vi "CalibrateCameraHeight (Standalone).vi"(0 "Inputs: Collect Images":T4={"Image feed"=refnum, "Axes Speeds [mm/s]"={"X Speed"=10.0, "Y Speed"=10.0, "Z Speed"=10.0}, "XYZ .NET Refnum in"=refnum}, 2 "Autofocus Coordinates":T3, 3 "Focusing test range [mm]":dbl, 4 "Stepsize [mm]":dbl, 5 "error in (no error)":errorcluster, 8 "Path to save collected images":path=path "E:/XYZstage+Camera_CollectedImages/12-17-2016/images") -> (14 "Optimized working distance [mm]":dbl, 15 "Uncertainty on optimized Z [mm]":dbl, 19 "error out":errorcluster)   [LabVIEW 2016]
uses:
  C:/Users/Aerotech/Documents/BNLStaveAssembly-blueprint/Bin/Aerotech.A3200.dll
  BNLStaveAssembly-blueprint/Bin/Aerotech.A3200.dll
  <vilib>/userdefined/High Color/IMAQdx.ctl
  <vilib>/vision/Image Controls.llb/IMAQ Image.ctl
  AerotechLibraries/Motion/EnableMultiple.vi
  <vilib>/vision/driver/NI_Vision_Acquisition_Software.lvlib
panel:
  in  "Wait time before \nimage capture [s]":dbl=3.5
  out "Wait to capture [ms]":u32=3500
  out "VISA error out":errorcluster
  out "double( Time, Temp )":dbl[](array[numeric])
  in  "stop":bool
  out "Camera error out":errorcluster
  in  "Camera gain":dbl=16.0
  out "Current field of view":T1(plugin-control)
  in  "Camera Name":T2="cam1" caption="IMAQdx Session"
  in  "Tab Control":enum32{"Inputs", "Results", "Error handling"}(tab)
  in  "Si Gain":dbl=9.5 format="%#_13g"
  in  "Spotlight":bool
  in  "Stave Gain":dbl=16.0 format="%#_13g"
  # "CALIBRATE CAMERA HEIGHT Brandeis University - Brookhaven National Laboratory * ATLAS Phase II Inner Tracker Upgrade"
types:
  T1 = typedef "IMAQ Image.ctl" = refnum<image>
  T2 = typedef "IMAQdx.ctl" = refnum<k21>
  T3 = cluster{"Go to X":dbl, "Go to Y":dbl, "Go to Z":dbl}
  T4 = cluster{"Image feed":T1, "Axes Speeds [mm/s]":cluster{"X Speed":dbl, "Y Speed":dbl, "Z Speed":dbl}, "XYZ .NET Refnum in":refnum<k24>}
  T5 = typedef "Image Type" = u32
  T6 = cluster{"Captured positions":dbl[][], "XYZ .NET Refnum out":refnum<k24>}
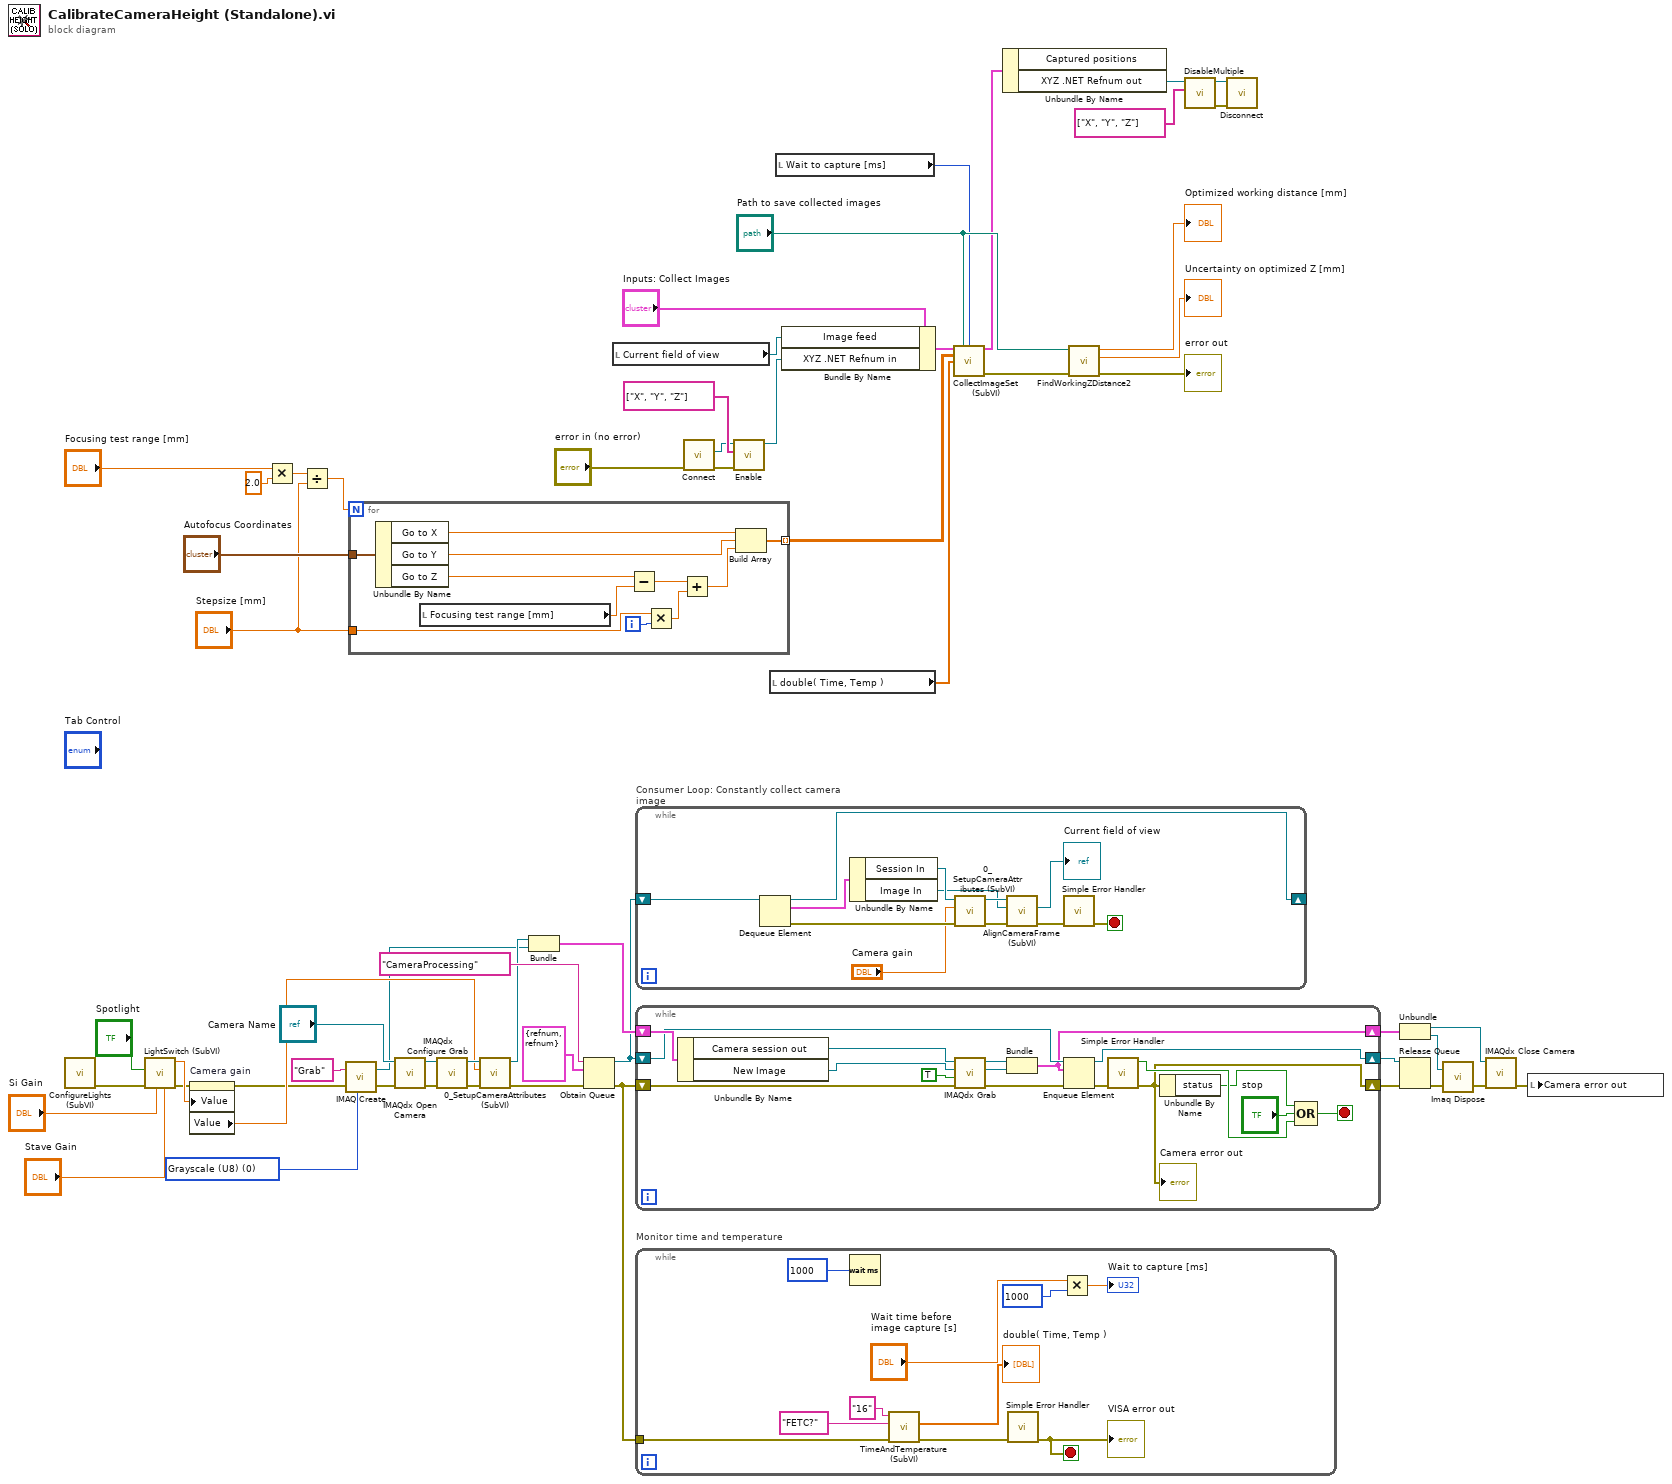
[diagram p0: block diagram]
diagram:
  w34 = T5 0 items=["Grayscale (U8)", "Grayscale (I16)", "Grayscale (SGL)", "Complex (CSG)", "RGB (U32)", "HSL (U32)", "RGB (U64)", "Grayscale (U16)"] ("Image Type")
  n1 = call "ConfigureLights (SubVI).vi"() -> ("error out"=w17:errorcluster)  [unwired: 11 in]
  n2 = call "LightSwitch (SubVI).vi"("Stave Gain"="Stave Gain", "Si Gain"="Si Gain", "error in"=w17, "Spotlight"="Spotlight") -> ("error out"=w26:errorcluster, "Assigned camera gain"=w27:dbl)  [unwired: 5 in, 1 out]
  n3 = property on="Camera gain" class="DigNum (strict)"(error in=w26, "Value"=w27) -> (error out=w16:errorcluster, "Value"=w21:dbl)  [unwired: 1 in, 1 out]
  n4 = Multiply(x="Focusing test range [mm]", y=2.0) -> (x*y=w54:dbl)
  n5 = Divide(x=w54, y="Stepsize [mm]") -> (x/y=w56:dbl)
  n6 = call "IMAQ Create"("Image Name"="Grab", "Image Type"=w34, "error in (no error)"=w16) -> ("New Image"=w18:T1, "error out"=w31:errorcluster)  [unwired: 1 in, 1 out]
  n7 = for {
    N: w56 -> [_]
    tunnel: "Autofocus Coordinates" -> [w70]
    tunnel: [w67] -> w58 mode=indexing
    tunnel: "Stepsize [mm]" -> [w65]
    i -> [w66]
    n8 = Unbundle By Name(w70) -> ("Go to X"=w69:dbl, "Go to Y"=w68:dbl, "Go to Z"=w64:dbl)
    n9 = local read "Focusing test range [mm]"() -> (w63:dbl)
    n10 = Subtract(x=w64, y=w63) -> (x-y=w62:dbl)
    n11 = Multiply(x=w65, y=w66) -> (x*y=w61:dbl)
    n12 = Add(x=w62, y=w61) -> (x+y=w60:dbl)
    n13 = Build Array(w69, w68, w60) -> (w67:dbl[])
  }
  n14 = call <vilib>:"IMAQdx Open Camera.vi"("error in"=w31, "Session In"="Camera Name") -> ("error out"=w32:errorcluster, "Session Out"=w35:T2)  [unwired: 1 in, 7 out]
  n15 = call <vilib>:"IMAQdx Configure Grab.vi"("error in"=w32, "Session In"=w35) -> ("error out"=w22:errorcluster, "Session Out"=w23:T2)  [unwired: 8 out]
  n16 = call "0_SetupCameraAttributes (SubVI).vi"("error in (no error)"=w22, "Gain"=w21, "Camera session in"=w23) -> ("error out"=w20:errorcluster, "Camera session out"=w19:T2)  [unwired: 7 in]
  n17 = Bundle("Camera session out"=w19, "New Image"=w18) -> (w12:cluster{"Camera session out":T2, "New Image":T1})  [unwired: 1 in]
  n18 = Obtain Queue(name (unnamed)="CameraProcessing", element data type=cluster{"Session In":T2, "Image In":T1} {"Session In"="", "Image In"=refnum}, error in (no error)=w20) -> (queue out=w10:refnum<queue>, error out=w3:errorcluster)  [unwired: 2 in, 1 out]
  n19 = local read "Current field of view"() -> (w5:T1)
  n20 = while "Consumer Loop: Constantly collect camera image" {
    shift-right: [w79] -> _
    shift-left: w10 -> [w82]
    stop <- w71 stop-if-true
    n21 = Dequeue Element(queue=w82) -> (queue out=w79:refnum<queue>, element=w81:cluster{"Session In":T2, "Image In":T1}, error out=w80:errorcluster)  [unwired: 2 in, 1 out]
    n22 = Unbundle By Name(w81) -> ("Session In"=w78:T2, "Image In"=w76:T1)
    n23 = call "0_SetupCameraAttributes (SubVI).vi"("error in (no error)"=w80, "Gain"="Camera gain", "Camera session in"=w78) -> ("error out"=w75:errorcluster, "Camera session out"=w77:T2)  [unwired: 7 in]
    n24 = call "AlignCameraFrame (SubVI).vi"("error in (no error)"=w75, "Image Src"=w76, "Camera session in"=w77) -> ("error out"=w72:errorcluster, "Image Dst Out"=→"Current field of view":T1)  [unwired: 6 in, 1 out]
    n25 = call <vilib>:"Simple Error Handler.vi"("error in (no error)"=w72) -> ("error out"=w71:errorcluster)  [unwired: 4 in, 4 out]
  }
  n26 = while {
    shift-right: [w89] -> w11
    shift-left: w10 -> [w88]
    shift-right: [w85] -> w9
    shift-left: w12 -> [w92]
    shift-right: [w83] -> w6
    shift-left: w3 -> [w84]
    stop <- w87 stop-if-true
    n27 = Unbundle By Name(w92) -> ("Camera session out"=w91:T2, "New Image"=w90:T1)
    n28 = call <vilib>:"IMAQdx Grab.vi"("error in"=w84, "Wait for Next Buffer? (Yes)"=TRUE, "Image In"=w90, "Session In"=w91) -> ("error out"=w98:errorcluster, "Image Out"=w94:T1, "Session Out"=w95:T2)  [unwired: 5 out]
    n29 = Bundle("Session Out"=w95, "Image Out"=w94) -> (w85:cluster{"Session Out":T2, "Image Out":T1})  [unwired: 1 in]
    n30 = Enqueue Element(queue=w88, element=w85, error in (no error)=w98) -> (queue out=w89:refnum<queue>, error out=w97:errorcluster)  [unwired: 1 in, 1 out]
    n31 = call <vilib>:"Simple Error Handler.vi"("error in (no error)"=w97) -> ("error?"=w99:bool, "error out"=w83:errorcluster)  [unwired: 4 in, 3 out]
    "Camera error out" <- w83
    n32 = Unbundle By Name(w83) -> ("status"=w96:bool)
    n33 = Compound Arithmetic op=OR(w96, "stop", w99) -> (w87:bool)
  }
  n34 = while "Monitor time and temperature" {
    tunnel: w3 -> [w106]
    stop <- w100 stop-if-true
    n35 = Wait (ms)(milliseconds to wait=u32 1000) -> ()  [unwired: 1 out]
    n36 = call "TimeAndTemperature (SubVI).vi"("error in (no error)"=w106, "Command"="FETC?", "GPIB Address: Temperature"="16") -> ("error out"=w101:errorcluster, "double( Time, Temp )"=→"double( Time, Temp )":dbl[])  [unwired: 5 in, 2 out]
    n37 = call <vilib>:"Simple Error Handler.vi"("error in (no error)"=w101) -> ("error out"=w100:errorcluster)  [unwired: 4 in, 4 out]
    "VISA error out" <- w100
    n38 = Multiply(x="Wait time before \nimage capture [s]", y=u32 1000) -> (x*y=→"Wait to capture [ms]":dbl)
  }
  n39 = call "Connect.vi"("error in (no error)"="error in (no error)") -> ("error out"=w46:errorcluster, "controller"=w44:refnum<k24>)  [unwired: 9 in]
  n40 = call-poly "Enable.vi"("error in (no error)"=w46, "axis names"=string[] ["X", "Y", "Z"], "controller in"=w44) -> ("controller out"=w42:refnum<k24>)  [unwired: 7 in, 1 out]
  n41 = local read "double( Time, Temp )"() -> (w2:dbl[])
  n42 = local read "Wait to capture [ms]"() -> (w1:u32)
  n43 = Bundle By Name(cluster="Inputs: Collect Images", "Image feed"=w5, "XYZ .NET Refnum in"=w42) -> (w4:T4)
  n44 = call "CollectImageSet (SubVI).vi"("Inputs"=w4, "Path to save collected images"="Path to save collected images", "milliseconds to wait"=w1, "Set of coordinates to process"=w58, "Time & Temperature Stamp"=w2) -> ("Outputs"=w41:T6, "error out"=w52:errorcluster)  [unwired: 8 in, 1 out]
  n45 = Unbundle By Name(w41) -> ("XYZ .NET Refnum out"=w38:refnum<k24>)  [unwired: 1 out]
  n46 = call "FindWorkingZDistance2.vi"("error in"=w52, "Images Directory"="Path to save collected images") -> ("error out"=→"error out":errorcluster, "Uncertainty on optimized Z"=→"Uncertainty on optimized Z [mm]":dbl, "Optimized Z"=→"Optimized working distance [mm]":dbl)  [unwired: 7 in]
  n47 = call "DisableMultiple.vi"("axis names"=string[] ["X", "Y", "Z"], "controller in"=w38) -> ("error out"=w40:errorcluster, "controller out"=w39:refnum<k24>)  [unwired: 8 in]
  n48 = call "Disconnect.vi"("error in (no error)"=w40, "controller"=w39) -> ()  [unwired: 9 in, 1 out]
  n49 = Unbundle(w9) -> ("Camera session out"=w7:T2, "New Image"=w8:T1)
  n50 = Release Queue(queue=w11, error in (no error)=w6) -> (error out=w14:errorcluster)  [unwired: 1 in, 2 out]
  n51 = call "Imaq Dispose"("Image"=w8, "error in (no error)"=w14) -> ("error out"=w15:errorcluster)  [unwired: 4 in]
  n52 = call <vilib>:"IMAQdx Close Camera.vi"("error in"=w15, "Session In"=w7) -> ("error out"=w13:errorcluster)  [unwired: 9 in]
  n53 = local write "Camera error out"(w13) -> ()
